vi "Controle_Manip_Main_GUI_WorkingBackup_211222.vi"() -> ()   [LabVIEW 2019] (continued)
                                n1610 = local write "CCD 2D Image Main"(w2024) -> ()
                                }
                                }
                                }
                                }
                              }
                              frame True {
                              }
                            }
                          }
                          frame #1 {
                            # "measurement"
                            n1611 = local read "ESP 301 On?"() -> (w2048:bool)
                            n1612 = case shown="True" w2048 {
                              frame False {
                                n1613 = local read "Log file"() -> (w2052:string)
                                n1614 = call "Write2LogFile.vi"("Add to log file"="ESP301 not activated", "Log file before"=w2052, "Checkbox"=FALSE) -> ("Log file after"=w2051:string)
                                n1615 = local write "Log file"(w2051) -> ()
                              }
                              frame True {
                                n1616 = stacked-sequence {
                                frame #0 {
                                # "get refs and exp params"
                                n1617 = local read "LightField Automation out"() -> (w2063:refnum<class "LightField Automation.lvclass">)
                                n1618 = local read "Photodiode error out"() -> (w2058:errorcluster)
                                n1619 = local read "LightField Automation error out"() -> (w2062:errorcluster)
                                n1620 = local read "ESP 301 COM Port"() -> (w2061:refnum<visa-resource-name>)
                                n1621 = local read "Photodiode handle out"() -> (w2059:refnum<visa-resource-name>)
                                n1622 = local read "ESP 301 Error"() -> (w2060:errorcluster)
                                n1623 = property on="Full scale" class="Bool (strict)"("Val(Sgnl)"=TRUE ("Value (Signaling)")) -> ()  [unwired: 2 in, 2 out]
                                n1624 = Bundle("LightField Automation out"=w2063, "LightField Automation error out"=w2062, "ESP 301 COM Port"=w2061, "ESP 301 Error"=w2060, "Photodiode handle out"=w2059, "Photodiode error out"=w2058) -> (→"Test Handles Polar":T16)  [unwired: 1 in]
                                n1625 = local read "CCD ROI"() -> (w2054:T20)
                                n1626 = local read "Exposure Time (ms)"() -> (w2065:dbl)
                                n1627 = local read "Polar Start Angle (°)"() -> (w2069:dbl)
                                n1628 = local read "Polar Step Angle (°)"() -> (w2068:dbl)
                                n1629 = local read "Polar End Angle (°)"() -> (w2064:dbl)
                                n1630 = local read "KCube Shutter On?"() -> (w2057:bool)
                                n1631 = local read "Polar mode"() -> (w2066:u16)
                                n1632 = local read "Acq Mode"() -> (w2067:T3)
                                n1633 = Bundle("Polar End Angle (°)"=w2064, "Polar Start Angle (°)"=w2069, "Polar Step Angle (°)"=w2068, "Acq Mode"=w2067, "Polar mode"=w2066, "Exposure Time (ms)"=w2065, "CCD ROI"=w2054, "KCube Shutter On?"=w2057) -> (→"Polar Params SubVIv2":T15)  [unwired: 1 in]
                                }
                                frame #1 {
                                # "Prepare graph and controls"
                                n1634 = local read "Scan Polarisation References"() -> (w2073:T17)
                                n1635 = local read "Polar Params SubVIv2"() -> (w2074:T15)
                                n1636 = local read "Scan Polar Params"() -> (w2075:refnum<vi>[])
                                n1637 = call "SubVI_PrePolarisation.vi"("Test References"=w2073, "Polar Params SubVIv2"=w2074, "Scan Polar Params"=w2075) -> ()
                                n1638 = property on="Elapsed (s)" class="DigNum (strict)"("Visible"=TRUE) -> ()  [unwired: 2 in, 2 out]
                                n1639 = property on="CCD 1D Spectrum Main" class="XYGraph (strict)"() -> ("XScale.Maximum"=w2078:dbl, "XScale.Minimum"=w2077:dbl, "YScale.Minimum"=w2072:dbl, "YScale.Maximum"=w2076:dbl)  [unwired: 2 in, 2 out]
                                n1640 = property on="Experiment Graph Controls" class="TabCtl (strict)"("Value"=T25."Polar" ("Experiment Graph Controls")) -> ()  [unwired: 2 in, 2 out]
                                n1641 = property on="Polarisation 1D Spectrum" class="XYGraph (strict)"("XScale.Maximum"=w2078, "XScale.Minimum"=w2077, "YScale.Minimum"=w2072, "YScale.Maximum"=w2076) -> ()  [unwired: 2 in, 2 out]
                                }
                                frame #2 {
                                # "actual exp"
                                n1642 = local read "Scan Polarisation References"() -> (w2085:T17)
                                n1643 = local read "Polar Params SubVIv2"() -> (w2086:T15)
                                n1644 = local read "Test Handles Polar"() -> (w2084:T16)
                                n1645 = call "Polarisation_v2.vi"("Test Handles Polar"=w2084, "Polar Params SubVIv2"=w2086, "Test References"=w2085) -> ("2D Pol Data"=w2083:dbl[][], "Test Handles Out"=w2081:T35, "Angles"=w2082:dbl[], "Wavelengths"=w2079:dbl[], "Puissances"=→"PuissancesPolar":dbl[])  [unwired: 1 in]
                                n1646 = local write "Test Handles Polar"(w2081) -> ()
                                n1647 = local write "Angles"(w2082) -> ()
                                n1648 = local write "Wavelength calibration"(w2079) -> ()
                                n1649 = local write "Pol 2D Array Out"(w2083) -> ()
                                }
                                frame #3 {
                                n1650 = control-ref of="MasterStop"() -> (w2088:refnum<vi>)
                                n1651 = control-ref of="MasterPause"() -> (w2089:refnum<vi>)
                                n1652 = control-ref of="ExperimentStopped?"() -> (w2087:refnum<vi>)
                                n1653 = call "CheckStopAndReset.vi"("ExperimentStopped?"=w2087, "MasterStop"=w2088, "MasterPause"=w2089) -> ()
                                }
                                frame #4 {
                                # "end exp"
                                n1654 = local read "Scan Polarisation References"() -> (w2095:T17)
                                n1655 = local read "Scan Polar Params"() -> (w2096:refnum<vi>[])
                                n1656 = local read "Angles"() -> (w2097:dbl[])
                                n1657 = local read "Test Handles Polar"() -> (w2094:T16)
                                n1658 = call "SubVI_PostPolarisation.vi"("Test References"=w2095, "Angles"=w2097, "Scan Polar Params"=w2096) -> ()
                                n1659 = Unbundle By Name(w2094) -> ("LightField Automation out"=w2093:refnum<class "LightField Automation.lvclass">, "LightField Automation error out"=w2092:errorcluster)
                                n1660 = property on="Elapsed (s)" class="DigNum (strict)"("Visible"=FALSE) -> ()  [unwired: 2 in, 2 out]
                                n1661 = local write "LightField Automation error out"(w2092) -> ()
                                n1662 = local write "LightField Automation out"(w2093) -> ()
                                n1663 = property on="Experiment Graph Controls" class="TabCtl (strict)"("Value"=T25."Polar" ("Experiment Graph Controls")) -> ()  [unwired: 2 in, 2 out]
                                }
                                }
                              }
                            }
                          }
                        }
                      }
                      frame "Acquire Contrast" {
                        n1664 = stacked-sequence {
                          frame #0 {
                            # "background"
                            n1665 = local read "Background taken?"() -> (w2098:bool)
                            n1666 = case shown="False" w2098 {
                              frame False {
                                n1667 = stacked-sequence {
                                tunnel: [_ _ w2148] -> w2099
                                frame #0 {
                                n1668 = local read "Log file"() -> (w2133:string)
                                n1669 = property on="CCD 1D Spectrum Main" class="XYGraph (strict)"("YScale.Offset"=0.0 ("Y Scale.Offset and Multiplier:Offset")) -> ()  [unwired: 2 in, 2 out]
                                n1670 = call "Write2LogFile.vi"("Add to log file"="Acquiring background", "Log file before"=w2133, "Checkbox"=FALSE) -> ("Log file after"=w2132:string)
                                n1671 = local write "Log file"(w2132) -> ()
                                }
                                frame #1 {
                                # "make sure shutter is closed"
                                n1672 = local read "KCube Shutter On?"() -> (w2134:bool)
                                n1673 = control-ref of="Shutter Ctrls"() -> (w2138:refnum<vi>)
                                n1674 = property class="Ring (strict)"(reference=w2138) -> ("Value"=w2137:u16)  [unwired: 1 in, 2 out]
                                n1675 = control-ref of="KCube Shutter Device Reference"() -> (w2139:refnum<vi>)
                                n1676 = Equal?(x=w2137, y=u16 0) -> (x = y?=w2135:bool)
                                n1677 = case shown="False" w2135 {
                                tunnel: w2139 -> [w2142 _]
                                tunnel: w2138 -> [w2141 _]
                                tunnel: w2134 -> [w2140 _]
                                frame False {
                                n1678 = call "Shutter.vi"("KCube Shutter Device Reference 2"=w2142, "Shutter Ctrls 2"=w2141, "Shutter on?"=w2140) -> ()
                                }
                                frame True {
                                }
                                }
                                }
                                frame #2 {
                                # "acquire"
                                n1679 = local read "LightField Automation error out"() -> (w2146:errorcluster)
                                n1680 = local read "LightField Automation out"() -> (w2147:refnum<class "LightField Automation.lvclass">)
                                n1681 = local read "Accumulations"() -> (w2143:dbl)
                                n1682 = call "LFA_Capture.vi"("error in (no error)"=w2146, "Frames"=w2143, "LightField Automation in"=w2147) -> ("error out"=w2145:errorcluster, "Data"=w2148:T26, "LightField Automation out"=w2144:refnum<class "LightField Automation.lvclass">)  [unwired: 6 in]
                                n1683 = local write "LightField Automation error out"(w2145) -> ()
                                n1684 = local write "LightField Automation out"(w2144) -> ()
                                }
                                }
                                n1685 = local read "Acq Mode"() -> (w2100:T3)
                                n1686 = case shown="\"Spectrum\", Default" w2100 {
                                selector: w2100 -> [w2101 w2119]
                                tunnel: w2099 -> [w2102 w2120]
                                frame "Spectrum", Default {
                                n1687 = stacked-sequence {
                                tunnel: w2102 -> [_ w2113 _ _]
                                tunnel: w2101 -> [_ w2111 _ _]
                                frame #0 {
                                n1688 = property on="CCD 2D Image Main" class="IntGraph (strict)"("Visible"=FALSE) -> ()  [unwired: 2 in, 2 out]
                                n1689 = property on="CCD 1D Spectrum Main" class="XYGraph (strict)"("Visible"=TRUE) -> ()  [unwired: 2 in, 2 out]
                                }
                                frame #1 {
                                n1690 = local read "Wavelength calibration"() -> (w2110:dbl[])
                                n1691 = local read "CCD ROI"() -> (w2106:T20)
                                n1692 = Divide(x=1239.842, y=w2110) -> (x/y=w2108:dbl[])
                                n1693 = call "PrepareData4Graph.vi"("Wavelength nm"=w2108, "DataLF"=w2113, "CCD ROI"=w2106, "AcqMode"=w2111, "Data type"=T30."Spectre") -> ("Spectrum"=w2112:cluster{"Array 2":dbl[], "Array":dbl[]}, "PLInt out"=w2105:dbl[])  [unwired: 2 in, 2 out]
                                n1694 = local write "CCD 1D Spectrum Main"(w2112) -> ()
                                n1695 = local write "BackgroundSpec"(w2105) -> ()
                                }
                                frame #2 {
                                n1696 = local read "BackgroundSpec"() -> (w2114:dbl[])
                                n1697 = call-poly <vilib>:"Mean.vi"("X"=w2114) -> ("mean"=w2116:dbl)  [unwired: 1 out]
                                n1698 = Negate(x=w2116) -> (-x=w2115:dbl)
                                n1699 = property on="CCD 1D Spectrum Main" class="XYGraph (strict)"("YScale.Offset"=w2115) -> ()  [unwired: 2 in, 2 out]
                                }
                                frame #3 {
                                n1700 = local write "Background taken?"(TRUE ("Background taken?")) -> ()
                                n1701 = property on="Background substract" class="Enum (strict)"("Value"=enum16{"None", "Shutter"}."None" ("Background substract")) -> ()  [unwired: 2 in, 2 out]
                                }
                                }
                                }
                                frame "Image" {
                                n1702 = stacked-sequence {
                                tunnel: w2120 -> [_ w2128]
                                tunnel: w2119 -> [_ w2126]
                                frame #0 {
                                n1703 = property on="CCD 1D Spectrum Main" class="XYGraph (strict)"("Visible"=FALSE) -> ()  [unwired: 2 in, 2 out]
                                n1704 = property on="CCD 2D Image Main" class="IntGraph (strict)"("Visible"=TRUE) -> ()  [unwired: 2 in, 2 out]
                                }
                                frame #1 {
                                n1705 = local read "Wavelength calibration"() -> (w2127:dbl[])
                                n1706 = local read "CCD ROI"() -> (w2123:T20)
                                n1707 = call "PrepareData4Graph.vi"("Wavelength nm"=w2127, "DataLF"=w2128, "CCD ROI"=w2123, "AcqMode"=w2126, "Data type"=T30."Spectre") -> ("Intensity Graph"=w2125:dbl[][])  [unwired: 2 in, 3 out]
                                n1708 = local write "CCD 2D Image Main"(w2125) -> ()
                                }
                                }
                                }
                                }
                              }
                              frame True {
                              }
                            }
                          }
                          frame #1 {
                            # "measurement"
                            n1709 = stacked-sequence {
                              frame #0 {
                                w2151 = FALSE ("Value")
                                w2152 = TRUE ("Visible")
                                w2156 = FALSE
                                w2161 = FALSE ("Acq Cont")
                                n1710 = property on="CCD 1D Spectrum Main" class="XYGraph (strict)"() -> ("XScale.Maximum"=w2160:dbl, "XScale.Minimum"=w2159:dbl, "YScale.Minimum"=w2158:dbl, "YScale.Maximum"=w2157:dbl)  [unwired: 2 in, 2 out]
                                n1711 = property on="Acquire Contrast" class="Bool (strict)"("Visible"=w2156) -> ()  [unwired: 2 in, 2 out]
                                n1712 = property on="Save Contrast" class="Bool (strict)"("Visible"=w2156) -> ()  [unwired: 2 in, 2 out]
                                n1713 = property on="Contrast 1D Spectrum" class="XYGraph (strict)"("XScale.Maximum"=w2160, "XScale.Minimum"=w2159, "YScale.Minimum"=w2158, "YScale.Maximum"=w2157) -> ()  [unwired: 2 in, 2 out]
                                n1714 = local read "Scan Contrast Ctrls"() -> (w2164:refnum<vi>[])
                                n1715 = property on="Scan Linear Stage Progess Bar" class="Slide (strict)"("Visible"=TRUE, "Value"=u8 0 ("Scan Linear Stage Progess Bar")) -> ()  [unwired: 2 in, 2 out]
                                n1716 = local write "Acquire Contrast"(w2161) -> ()
                                n1717 = local write "Save Contrast"(w2161) -> ()
                                n1718 = call "Enable&Disable_Controls.vi"("Enum"=enum16{"Enabled", "Disabled", "Disabled&Grayed"}."Disabled&Grayed", "References"=w2164) -> ()  [unwired: 1 in]
                                n1719 = property on="Scan Linear Stage Progess Bar" class="Slide (strict)"("Visible"=TRUE) -> ()  [unwired: 2 in, 2 out]
                                n1720 = property on="Elapsed (s)" class="DigNum (strict)"("Visible"=TRUE) -> ()  [unwired: 2 in, 2 out]
                                n1721 = control-ref of="MasterStop"() -> (w2154:refnum<vi>)
                                n1722 = control-ref of="MasterPause"() -> (w2153:refnum<vi>)
                                n1723 = property on="Experiment Graph Controls" class="TabCtl (strict)"("Value"=T25."Contrast" ("Experiment Graph Controls")) -> ()  [unwired: 2 in, 2 out]
                                n1724 = property class="Bool (strict)"(reference=w2153, "Visible"=w2152, "Value"=w2151) -> ()  [unwired: 1 in, 2 out]
                                n1725 = property class="Bool (strict)"(reference=w2154, "Visible"=w2152, "Value"=w2151) -> ()  [unwired: 1 in, 2 out]
                              }
                              frame #1 {
                                n1726 = local read "Excitation Wavelength (nm)"() -> (w2170:dbl)
                                n1727 = local read "LinTFines Step Pos (usteps)"() -> (w2175:dbl)
                                n1728 = local read "LinTFine Start Pos (usteps)"() -> (w2176:dbl)
                                n1729 = local read "LinTFine End Pos (usteps)"() -> (w2174:dbl)
                                n1730 = local read "Exposure Time (ms)"() -> (w2172:dbl)
                                n1731 = local read "LinT Start Pos (mm)"() -> (w2179:dbl)
                                n1732 = local read "LinT Step Pos (mm)"() -> (w2178:dbl)
                                n1733 = local read "LinT End pos (mm)"() -> (w2177:dbl)
                                n1734 = local read "KCube Shutter On?"() -> (w2167:bool)
                                n1735 = local read "Accumulations"() -> (w2171:dbl)
                                n1736 = local read "Acq Mode"() -> (w2169:T3)
                                n1737 = local read "CCD ROI"() -> (w2168:T20)
                                n1738 = Bundle("LinT Start Pos (mm)"=w2179, "LinT Step Pos (mm)"=w2178, "LinT End pos (mm)"=w2177, "LinTFine Start Pos (usteps)"=w2176, "LinTFines Step Pos (usteps)"=w2175, "LinTFine End Pos (usteps)"=w2174) -> (w2173:T27)  [unwired: 1 in]
                                n1739 = Bundle("Exposure Time (ms)"=w2172, "Accumulations"=w2171, "Excitation Wavelength (nm)"=w2170, "Acq Mode"=w2169, "CCD ROI"=w2168, "KCube Shutter On?"=w2167) -> (w2166:T24)  [unwired: 1 in]
                                n1740 = local write "Scan Translation Params"(w2173) -> ()
                                n1741 = local write "Scan Translation Exp Params"(w2166) -> ()
                              }
                              frame #2 {
                                n1742 = local read "Scan Translation Exp Params"() -> (w2187:T24)
                                n1743 = local read "Scan Translation Params"() -> (w2204:T27)
                                n1744 = control-ref of="Scan Linear Stage Progess Bar"() -> ()  [unwired: 1 out]
                                n1745 = control-ref of="Stop Contrast"() -> ()  [unwired: 1 out]
                                n1746 = local read "ESP 301 COM Port"() -> (w2197:refnum<visa-resource-name>)
                                n1747 = control-ref of="Pause Contrast"() -> ()  [unwired: 1 out]
                                n1748 = control-ref of="Scan Main Progess Bar"() -> (w2186:refnum<vi>)
                                n1749 = local read "LightField Automation error out"() -> (w2184:errorcluster)
                                n1750 = local read "ESP 301 Error"() -> (w2199:errorcluster)
                                n1751 = local read "LightField Automation out"() -> (w2185:refnum<class "LightField Automation.lvclass">)
                                n1752 = control-ref of="Shutter Ctrls"() -> (w2189:refnum<vi>)
                                n1753 = control-ref of="KCube Shutter Device Reference"() -> (w2190:refnum<vi>)
                                n1754 = control-ref of="PZC Position Readout (usteps)"() -> (w2188:refnum<vi>)
                                n1755 = control-ref of="Contrast 1D Spectrum"() -> (w2191:refnum<vi>)
                                n1756 = control-ref of="Contrast Oscillations"() -> (w2192:refnum<vi>)
                                n1757 = Open VI Reference(type specifier VI Refnum (for type only)=refnum<vi> refnum ("application reference (local)"), vi path=path "C:/Users/manip/Documents/Controle_Manip_2020/subVIs/Scans/FineContrast_cleaned inputs.vi", options=256) -> (vi reference=w2202:refnum<vi>, error out=w2211:errorcluster)  [unwired: 3 in]
                                n1758 = local read "PZC200 Instrument Channel"() -> (w2203:string)
                                n1759 = call-by-ref "Wait On Asynchronous Call"(reference=w2202, error in=w2211) -> (reference out=w2210:refnum<vi>, error out=w2209:errorcluster, "PZAPos & InstPow"=w2200:dbl[][], "Spectra vs PZA"=w2207:i32[][], "LFA out"=w2183:refnum<class "LightField Automation.lvclass">, "PZC out"=w2201:string, "Photodiode out"=w2193:refnum<visa-resource-name>, "ESP 301 COM out"=w2196:refnum<visa-resource-name>, "LFA error out"=w2182:errorcluster, "PZC error out"=w2194:errorcluster, "Photodiode error out"=w2195:errorcluster, "ESP 301 error out"=w2198:errorcluster)  [unwired: 18 in]
                                n1760 = local write "PZAPos&Pow"(w2200) -> ()
                                n1761 = local write "Photodiode error out"(w2195) -> ()
                                n1762 = local write "PZC200 Instrument Channel"(w2201) -> ()
                                n1763 = local write "Contrast Array Out"(w2207) -> ()
                                n1764 = local read "PZC Error"() -> (w2208:errorcluster)
                                n1765 = local write "ESP 301 COM Port"(w2196) -> ()
                                n1766 = Close Reference(reference=w2210, error in (no error)=w2209) -> ()  [unwired: 1 out]
                                n1767 = local write "Photodiode handle out"(w2193) -> ()
                                n1768 = local read "Photodiode handle out"() -> (w2205:refnum<visa-resource-name>)
                                n1769 = local write "ESP 301 Error"(w2198) -> ()
                                n1770 = local read "Photodiode error out"() -> (w2206:errorcluster)
                                n1771 = local write "LightField Automation error out"(w2182) -> ()
                                n1772 = local write "LightField Automation out"(w2183) -> ()
                                n1773 = local write "PZC Error"(w2194) -> ()
                                n1774 = control-ref of="MasterStop"() -> (w2180:refnum<vi>)
                                n1775 = control-ref of="MasterPause"() -> (w2181:refnum<vi>)
                                n1776 = call-by-ref "Start Asynchronous Call"(reference=w2202, error in=w2211, "LFA in"=w2185, "PZC in"=w2203, "Photodiode in"=w2205, "ESP 301 COM"=w2197, "LFA error in"=w2184, "PZC error in"=w2208, "Photodiode error in"=w2206, "ESP 301 error in"=w2199, "Scan Translation Exp Params"=w2187, "PZC Pos (usteps)"=w2188, "Scan Translation Params"=w2204, "Pause button"=w2181, "Contrast Oscillations"=w2192, "Stop button"=w2180, "Contrast 1D Spectrum"=w2191, "Progess Bar"=w2186, "Shutter Device"=w2190, "Shutter"=w2189) -> ()  [unwired: 12 out]
                              }
                              frame #3 {
                                w2227 = FALSE ("Acq Cont")
                                w2224 = FALSE ("Acq Cont")
                                n1777 = local read "Auto< ?"() -> (w2222:bool)
                                n1778 = property on="Scan Linear Stage Progess Bar" class="Slide (strict)"("Visible"=FALSE, "Value"=u8 0 ("Scan Linear Stage Progess Bar")) -> ()  [unwired: 2 in, 2 out]
                                n1779 = Not(x=w2222) -> (.not. x?=w2221:bool)
                                n1780 = local write "Pause Michelson"(w2227) -> ()
                                n1781 = local write "Stop Michelson"(w2227) -> ()
                                n1782 = property on="Save Contrast" class="Bool (strict)"("Visible"=w2221) -> ()  [unwired: 2 in, 2 out]
                                n1783 = property on="Acquire Contrast" class="Bool (strict)"("Visible"=TRUE) -> ()  [unwired: 2 in, 2 out]
                                n1784 = local write "Acquire Michelson"(w2224) -> ()
                                n1785 = local write "Acquire Contrast"(w2224) -> ()
                                n1786 = local write "Save Michelson"(w2224) -> ()
                                n1787 = local read "Scan Contrast Ctrls"() -> (w2220:refnum<vi>[])
                                n1788 = property on="Elapsed (s)" class="DigNum (strict)"("Visible"=FALSE) -> ()  [unwired: 2 in, 2 out]
                                n1789 = control-ref of="MasterStop"() -> (w2217:refnum<vi>)
                                n1790 = control-ref of="MasterPause"() -> (w2218:refnum<vi>)
                                n1791 = call "Enable&Disable_Controls.vi"("Enum"=enum16{"Enabled", "Disabled", "Disabled&Grayed"}."Enabled", "References"=w2220) -> ()  [unwired: 1 in]
                                n1792 = control-ref of="ExperimentStopped?"() -> (w2216:refnum<vi>)
                                n1793 = call "CheckStopAndReset.vi"("ExperimentStopped?"=w2216, "MasterStop"=w2217, "MasterPause"=w2218) -> ()
                              }
                            }
                          }
                        }
                      }
                      frame "Acquire Michelson" {
                        n1794 = stacked-sequence {
                          frame #0 {
                            # "background"
                            n1795 = local read "Background taken?"() -> (w2228:bool)
                            n1796 = case shown="False" w2228 {
                              frame False {
                                n1797 = stacked-sequence {
                                tunnel: [_ _ w2278] -> w2229
                                frame #0 {
                                n1798 = local read "Log file"() -> (w2263:string)
                                n1799 = property on="CCD 1D Spectrum Main" class="XYGraph (strict)"("YScale.Offset"=0.0 ("Y Scale.Offset and Multiplier:Offset")) -> ()  [unwired: 2 in, 2 out]
                                n1800 = call "Write2LogFile.vi"("Add to log file"="Acquiring background", "Log file before"=w2263, "Checkbox"=FALSE) -> ("Log file after"=w2262:string)
                                n1801 = local write "Log file"(w2262) -> ()
                                }
                                frame #1 {
                                # "make sure shutter is closed"
                                n1802 = local read "KCube Shutter On?"() -> (w2264:bool)
                                n1803 = control-ref of="Shutter Ctrls"() -> (w2268:refnum<vi>)
                                n1804 = property class="Ring (strict)"(reference=w2268) -> ("Value"=w2267:u16)  [unwired: 1 in, 2 out]
                                n1805 = control-ref of="KCube Shutter Device Reference"() -> (w2269:refnum<vi>)
                                n1806 = Equal?(x=w2267, y=u16 0) -> (x = y?=w2265:bool)
                                n1807 = case shown="False" w2265 {
                                tunnel: w2269 -> [w2272 _]
                                tunnel: w2268 -> [w2271 _]
                                tunnel: w2264 -> [w2270 _]
                                frame False {
                                n1808 = call "Shutter.vi"("KCube Shutter Device Reference 2"=w2272, "Shutter Ctrls 2"=w2271, "Shutter on?"=w2270) -> ()
                                }
                                frame True {
                                }
                                }
                                }
                                frame #2 {
                                # "acquire"
                                n1809 = local read "LightField Automation error out"() -> (w2276:errorcluster)
                                n1810 = local read "LightField Automation out"() -> (w2277:refnum<class "LightField Automation.lvclass">)
                                n1811 = local read "Accumulations"() -> (w2273:dbl)
                                n1812 = call "LFA_Capture.vi"("error in (no error)"=w2276, "Frames"=w2273, "LightField Automation in"=w2277) -> ("error out"=w2275:errorcluster, "Data"=w2278:T26, "LightField Automation out"=w2274:refnum<class "LightField Automation.lvclass">)  [unwired: 6 in]
                                n1813 = local write "LightField Automation error out"(w2275) -> ()
                                n1814 = local write "LightField Automation out"(w2274) -> ()
                                }
                                }
                                n1815 = local read "Acq Mode"() -> (w2230:T3)
                                n1816 = case shown="\"Spectrum\", Default" w2230 {
                                selector: w2230 -> [w2231 w2249]
                                tunnel: w2229 -> [w2232 w2250]
                                frame "Spectrum", Default {
                                n1817 = stacked-sequence {
                                tunnel: w2232 -> [_ w2243 _ _]
                                tunnel: w2231 -> [_ w2241 _ _]
                                frame #0 {
                                n1818 = property on="CCD 2D Image Main" class="IntGraph (strict)"("Visible"=FALSE) -> ()  [unwired: 2 in, 2 out]
                                n1819 = property on="CCD 1D Spectrum Main" class="XYGraph (strict)"("Visible"=TRUE) -> ()  [unwired: 2 in, 2 out]
                                }
                                frame #1 {
                                n1820 = local read "Wavelength calibration"() -> (w2240:dbl[])
                                n1821 = local read "CCD ROI"() -> (w2236:T20)
                                n1822 = Divide(x=1239.842, y=w2240) -> (x/y=w2238:dbl[])
                                n1823 = call "PrepareData4Graph.vi"("Wavelength nm"=w2238, "DataLF"=w2243, "CCD ROI"=w2236, "AcqMode"=w2241, "Data type"=T30."Spectre") -> ("Spectrum"=w2242:cluster{"Array 2":dbl[], "Array":dbl[]}, "PLInt out"=w2235:dbl[])  [unwired: 2 in, 2 out]
                                n1824 = local write "CCD 1D Spectrum Main"(w2242) -> ()
                                n1825 = local write "BackgroundSpec"(w2235) -> ()
                                }
                                frame #2 {
                                n1826 = local read "BackgroundSpec"() -> (w2244:dbl[])
                                n1827 = call-poly <vilib>:"Mean.vi"("X"=w2244) -> ("mean"=w2246:dbl)  [unwired: 1 out]
                                n1828 = Negate(x=w2246) -> (-x=w2245:dbl)
                                n1829 = property on="CCD 1D Spectrum Main" class="XYGraph (strict)"("YScale.Offset"=w2245) -> ()  [unwired: 2 in, 2 out]
                                }
                                frame #3 {
                                n1830 = local write "Background taken?"(TRUE ("Background taken?")) -> ()
                                n1831 = property on="Background substract" class="Enum (strict)"("Value"=enum16{"None", "Shutter"}."None" ("Background substract")) -> ()  [unwired: 2 in, 2 out]
                                }
                                }
                                }
                                frame "Image" {
                                n1832 = stacked-sequence {
                                tunnel: w2250 -> [_ w2258]
                                tunnel: w2249 -> [_ w2256]
                                frame #0 {
                                n1833 = property on="CCD 1D Spectrum Main" class="XYGraph (strict)"("Visible"=FALSE) -> ()  [unwired: 2 in, 2 out]
                                n1834 = property on="CCD 2D Image Main" class="IntGraph (strict)"("Visible"=TRUE) -> ()  [unwired: 2 in, 2 out]
                                }
                                frame #1 {
                                n1835 = local read "Wavelength calibration"() -> (w2257:dbl[])
                                n1836 = local read "CCD ROI"() -> (w2253:T20)
                                n1837 = call "PrepareData4Graph.vi"("Wavelength nm"=w2257, "DataLF"=w2258, "CCD ROI"=w2253, "AcqMode"=w2256, "Data type"=T30."Spectre") -> ("Intensity Graph"=w2255:dbl[][])  [unwired: 2 in, 3 out]
                                n1838 = local write "CCD 2D Image Main"(w2255) -> ()
                                }
                                }
                                }
                                }
                              }
                              frame True {
                              }
                            }
                          }
                          frame #1 {
                            # "measurement"
                            n1839 = Get Date/Time In Seconds() -> (seconds since 1Jan1904=w2279:timestamp)
                            n1840 = stacked-sequence {
                              tunnel: w2279 -> [_ _ w2313 w2437]
                              frame #0 {
                                w2285 = TRUE
                                w2286 = FALSE ("Acq Cont")
                                w2283 = TRUE
                                w2282 = FALSE
                                w2284 = FALSE
                                # "check that range is within translation stage travel"
                                # "get params and check feasability"
                                n1841 = property on="Save Michelson" class="Bool (strict)"("Visible"=w2284) -> ()  [unwired: 2 in, 2 out]
                                n1842 = property on="Pause Michelson" class="Bool (strict)"("Visible"=w2283) -> ()  [unwired: 2 in, 2 out]
                                n1843 = property on="Save Contrast" class="Bool (strict)"("Visible"=w2284) -> ()  [unwired: 2 in, 2 out]
                                n1844 = property on="Pause Contrast" class="Bool (strict)"("Visible"=w2283) -> ()  [unwired: 2 in, 2 out]
                                n1845 = property on="Stop Contrast" class="Bool (strict)"("Visible"=w2283) -> ()  [unwired: 2 in, 2 out]
                                n1846 = property on="Acquire Michelson" class="Bool (strict)"("Visible"=w2284) -> ()  [unwired: 2 in, 2 out]
                                n1847 = property on="Stop Michelson" class="Bool (strict)"("Visible"=w2283) -> ()  [unwired: 2 in, 2 out]
                                n1848 = property on="Acquire Contrast" class="Bool (strict)"("Visible"=w2284) -> ()  [unwired: 2 in, 2 out]
                                n1849 = property on="Scan Linear Stage Progess Bar" class="Slide (strict)"("Visible"=TRUE, "Value"=u8 0 ("Scan Linear Stage Progess Bar")) -> ()  [unwired: 2 in, 2 out]
                                n1850 = property on="Scan Michelson Progess Bar" class="Slide (strict)"("Value"=u8 0 ("Scan Michelson Progess Bar"), "Visible"=TRUE) -> ()  [unwired: 2 in, 2 out]
                                n1851 = local read "Scan Contrast Ctrls"() -> (w2292:refnum<vi>[])
                                n1852 = local write "Acquire Contrast"(w2286) -> ()
                                n1853 = local write "Save Contrast"(w2286) -> ()
                                n1854 = call "Enable&Disable_Controls.vi"("Enum"=enum16{"Enabled", "Disabled", "Disabled&Grayed"}."Disabled&Grayed", "References"=w2292) -> ()  [unwired: 1 in]
                                n1855 = property on="Michelson Expected (s)" class="DigNum (strict)"("Visible"=w2285) -> ()  [unwired: 2 in, 2 out]
                                n1856 = property on="Elapsed (s)" class="DigNum (strict)"("Visible"=TRUE) -> ()  [unwired: 2 in, 2 out]
                                n1857 = property on="Experiment Graph Controls" class="TabCtl (strict)"("Value"=T25."Contrast" ("Experiment Graph Controls")) -> ()  [unwired: 2 in, 2 out]
                                n1858 = property on="Michelson Elapsed (s)" class="DigNum (strict)"("Visible"=w2285) -> ()  [unwired: 2 in, 2 out]
                                n1859 = local write "Acquire Michelson"(w2282) -> ()
                                n1860 = local write "Save Michelson"(w2282) -> ()
                              }
                              frame #1 {
                                # "check that range is within translation stage travel"
                                # "get params"
                                n1861 = local read "Excitation Wavelength (nm)"() -> (w2297:dbl)
                                n1862 = local read "Exposure Time (ms)"() -> (w2299:dbl)
                                n1863 = local read "KCube Shutter On?"() -> (w2294:bool)
                                n1864 = local read "Accumulations"() -> (w2298:dbl)
                                n1865 = local read "Acq Mode"() -> (w2296:T3)
                                n1866 = local read "CCD ROI"() -> (w2295:T20)
                                n1867 = local read "LinTFines Step Pos (usteps)"() -> (w2302:dbl)
                                n1868 = local read "LinTFine Start Pos (usteps)"() -> (w2303:dbl)
                                n1869 = local read "LinTFine End Pos (usteps)"() -> (w2301:dbl)
                                n1870 = local read "LinT Start Pos (mm)"() -> (w2306:dbl)
                                n1871 = local read "LinT Step Pos (mm)"() -> (w2305:dbl)
                                n1872 = local read "LinT End pos (mm)"() -> (w2304:dbl)
                                n1873 = Bundle("Exposure Time (ms)"=w2299, "Accumulations"=w2298, "Excitation Wavelength (nm)"=w2297, "Acq Mode"=w2296, "CCD ROI"=w2295, "KCube Shutter On?"=w2294) -> (w2293:T24)  [unwired: 1 in]
                                n1874 = Bundle("LinT Start Pos (mm)"=w2306, "LinT Step Pos (mm)"=w2305, "LinT End pos (mm)"=w2304, "LinTFine Start Pos (usteps)"=w2303, "LinTFines Step Pos (usteps)"=w2302, "LinTFine End Pos (usteps)"=w2301) -> (w2300:T27)  [unwired: 1 in]
                                n1875 = local write "Scan Translation Exp Params"(w2293) -> ()
                                n1876 = local write "Scan Translation Params"(w2300) -> ()
                              }
                              frame #2 {
                                # "pzc & inst pow"
                                # "esp pos"
                                # "data"
                                # "move ESP"
                                n1877 = local read "LightField Automation out"() -> (w2310:refnum<class "LightField Automation.lvclass">)
                                n1878 = local read "ESP 301 COM Port"() -> (w2312:refnum<visa-resource-name>)
                                n1879 = local read "LinT Start Pos (mm)"() -> (w2323:dbl)
                                n1880 = local read "ESP 301 Error"() -> (w2319:errorcluster)
                                n1881 = local read "LinT Step Pos (mm)"() -> (w2324:dbl)
                                n1882 = local read "LinT End pos (mm)"() -> (w2328:dbl)
                                n1883 = local read "LinT Start Pos (mm)"() -> (w2329:dbl)
                                n1884 = local read "LinT Step Pos (mm)"() -> (w2326:dbl)
                                n1885 = local read "LightField Automation error out"() -> (w2309:errorcluster)
                                n1886 = Subtract(x=w2328, y=w2329) -> (x-y=w2327:dbl)
                                n1887 = Divide(x=w2327, y=w2326) -> (x/y=w2325:dbl)
                                n1888 = Increment(x=w2325) -> (x+1=w2322:dbl)
                                n1889 = for {
                                N: w2322 -> [w2335]
                                tunnel: w2324 -> [w2352]
                                tunnel: w2323 -> [w2351]
                                shift-right: [w2347] -> w2320
                                shift-left: dbl[] [] -> [w2348]
                                shift-right: [w2345] -> w2308
                                shift-left: w2310 -> [w2346]
                                shift-right: [w2343] -> w2307
                                shift-left: w2309 -> [w2344]
                                shift-right: [w2341] -> w2318
                                shift-left: w2319 -> [w2342]
                                shift-right: [w2339] -> w2316
                                shift-left: dbl[][][] [] -> [w2340]
                                shift-right: [w2337] -> w2314
                                shift-left: dbl[][][] [] -> [w2338]
                                tunnel: w2313 -> [w2333]
                                shift-right: [w2330] -> w2311
                                shift-left: w2312 -> [w2331]
                                i -> [w2334]
                                stop <- w2332 stop-if-true
                                # "ESP"
                                n1890 = Multiply(x=w2334, y=w2352) -> (x*y=w2350:dbl)
                                n1891 = Add(x=w2351, y=w2350) -> (x+y=w2349:dbl)
                                n1892 = Divide(x=w2334, y=w2335) -> (x/y=w2336:dbl)
                                n1893 = stacked-sequence {
                                tunnel: w2349 -> [w2357 w2363 _ _]
                                tunnel: w2348 -> [w2359 _ _ _]
                                tunnel: [w2358 _ _ _] -> w2347
                                tunnel: w2346 -> [_ _ w2406 _]
                                tunnel: [_ _ w2405 _] -> w2345
                                tunnel: w2344 -> [_ _ w2404 _]
                                tunnel: [_ _ w2403 _] -> w2343
                                tunnel: w2342 -> [w2356 _ _ _]
                                tunnel: [w2355 _ _ _] -> w2341
                                tunnel: w2340 -> [_ _ w2375 _]
                                tunnel: [_ _ w2373 _] -> w2339
                                tunnel: w2338 -> [_ _ w2372 _]
                                tunnel: [_ _ w2370 _] -> w2337
                                tunnel: w2336 -> [_ _ _ w2416]
                                tunnel: w2335 -> [_ _ _ w2415]
                                tunnel: w2334 -> [_ _ _ w2413]
                                tunnel: w2333 -> [_ _ _ w2414]
                                tunnel: [_ _ _ w2411] -> w2332
                                tunnel: w2331 -> [w2354 _ _ _]
                                tunnel: [w2353 _ _ _] -> w2330
                                frame #0 {
                                # "pos readout"
                                n1894 = control-ref of="Newport Linear Translation Stage Position Readout (mm)"() -> (w2360:refnum<vi>)
                                n1895 = call "ESP301_Go2Pos.vi"("VISA resource name"=w2354, "Set value"=w2357, "Axis (1)"=1, "Error In"=w2356, "DigNum Refnum"=w2360) -> ("VISA resource name 2"=w2353:refnum<visa-resource-name>, "Error In 2"=w2355:errorcluster)
                                n1896 = Insert Into Array(array=w2359, new element=w2357) -> (w2358:dbl[])  [unwired: 1 in]
                                }
                                frame #1 {
                                # "wait on ESP"
                                n1897 = Wait (ms)(milliseconds to wait=u32 50) -> ()  [unwired: 1 out]
                                n1898 = Number To Decimal String(number=w2363) -> (decimal integer string=w2366:string)  [unwired: 1 in]
                                n1899 = local read "Log file"() -> (w2369:string)
                                n1900 = Concatenate Strings("ESP moved to ", w2366) -> (w2365:string)
                                n1901 = call "Write2LogFile.vi"("Add to log file"=w2365, "Log file before"=w2369, "Checkbox"=FALSE) -> ("Log file after"=w2368:string)
                                n1902 = local write "Log file"(w2368) -> ()
                                }
                                frame #2 {
                                n1903 = control-ref of="Shutter Ctrls"() -> (w2393:refnum<vi>)
                                n1904 = control-ref of="Scan Linear Stage Progess Bar"() -> (w2389:refnum<vi>)
                                n1905 = control-ref of="KCube Shutter Device Reference"() -> (w2394:refnum<vi>)
                                n1906 = control-ref of="PZC Position Readout (usteps)"() -> (w2392:refnum<vi>)
                                n1907 = control-ref of="Pause Contrast"() -> (w2391:refnum<vi>)
                                n1908 = control-ref of="Contrast 1D Spectrum"() -> (w2395:refnum<vi>)
                                n1909 = control-ref of="Contrast Oscillations"() -> (w2396:refnum<vi>)
                                n1910 = local read "Photodiode handle out"() -> (w2385:refnum<visa-resource-name>)
                                n1911 = local read "Photodiode error out"() -> (w2386:errorcluster)
                                n1912 = control-ref of="Stop Contrast"() -> (w2390:refnum<vi>)
                                n1913 = local read "Scan Translation Params"() -> (w2398:T27)
                                n1914 = Open VI Reference(type specifier VI Refnum (for type only)=refnum<vi> refnum ("application reference (local)"), vi path=path "C:/Users/manip/Documents/Controle_Manip_2020/subVIs/Scans/FineContrast_cleaned inputs.vi", options=256) -> (vi reference=w2400:refnum<vi>, error out=w2399:errorcluster)  [unwired: 3 in]
                                n1915 = local read "Scan Translation Exp Params"() -> (w2397:T24)
                                n1916 = local read "PZC200 Instrument Channel"() -> (w2384:string)
                                n1917 = local read "ESP 301 Error"() -> (w2387:errorcluster)
                                n1918 = local read "PZC Error"() -> (w2383:errorcluster)
                                n1919 = local read "ESP 301 COM Port"() -> (w2388:refnum<visa-resource-name>)
                                n1920 = call-by-ref "Start Asynchronous Call"(reference=w2400, error in=w2399, "LFA in"=w2406, "PZC in"=w2384, "Photodiode in"=w2385, "ESP 301 COM"=w2388, "LFA error in"=w2404, "PZC error in"=w2383, "Photodiode error in"=w2386, "ESP 301 error in"=w2387, "Scan Translation Exp Params"=w2397, "PZC Pos (usteps)"=w2392, "Scan Translation Params"=w2398, "Pause button"=w2391, "Contrast Oscillations"=w2396, "Stop button"=w2390, "Contrast 1D Spectrum"=w2395, "Progess Bar"=w2389, "Shutter Device"=w2394, "Shutter"=w2393) -> ()  [unwired: 12 out]
                                n1921 = call-by-ref "Wait On Asynchronous Call"(reference=w2400, error in=w2399) -> ("PZAPos & InstPow"=w2371:dbl[][], "Spectra vs PZA"=w2374:i32[][], "LFA out"=w2405:refnum<class "LightField Automation.lvclass">, "PZC out"=w2380:string, "Photodiode out"=w2379:refnum<visa-resource-name>, "ESP 301 COM out"=w2381:refnum<visa-resource-name>, "LFA error out"=w2403:errorcluster, "PZC error out"=w2377:errorcluster, "Photodiode error out"=w2378:errorcluster, "ESP 301 error out"=w2382:errorcluster)  [unwired: 18 in, 2 out]
                                n1922 = local write "PZC200 Instrument Channel"(w2380) -> ()
                                n1923 = local write "Photodiode handle out"(w2379) -> ()
                                n1924 = local write "Photodiode error out"(w2378) -> ()
                                n1925 = local write "ESP 301 COM Port"(w2381) -> ()
                                n1926 = Insert Into Array(array=w2372, new element=w2371) -> (w2370:dbl[][][])  [unwired: 3 in]
                                n1927 = local write "ESP 301 Error"(w2382) -> ()
                                n1928 = local write "PZC Error"(w2377) -> ()
                                n1929 = Insert Into Array(array=w2375, new element=w2374) -> (w2373:dbl[][][])  [unwired: 3 in]
                                }
                                frame #3 {
                                n1930 = local read "Pause Michelson"() -> (w2410:bool)
                                n1931 = control-ref of="Expected (s)"() -> (w2408:refnum<vi>)
                                n1932 = Increment(x=w2413) -> (x+1=w2412:i32)
                                n1933 = Multiply(x=w2416, y=100.0) -> (x*y=w2418:dbl)
                                n1934 = call "Expectedtime.vi"("N"=w2415, "I"=w2412, "Reference time"=w2414) -> ("Expected time"=w2407:dbl, "Elapsed time"=w2409:dbl)
                                "Michelson Elapsed (s)" <- w2409
                                "Michelson Expected (s)" <- w2407
                                n1935 = property class="DigNum (strict)"(reference=w2408, "Value"=w2407) -> ()  [unwired: 1 in, 2 out]
                                n1936 = property on="Elapsed (s)" class="DigNum (strict)"("Value"=w2409) -> ()  [unwired: 2 in, 2 out]
                                n1937 = local write "Scan Michelson Progess Bar"(w2418) -> ()
                                n1938 = case shown="True" w2410 {
                                frame False {
                                }
                                frame True {
                                n1939 = while {
                                stop <- w2420 stop-if-true
                                n1940 = local read "Pause Michelson"() -> (w2421:bool)
                                n1941 = Wait (ms)(milliseconds to wait=u32 50) -> ()  [unwired: 1 out]
                                n1942 = Not(x=w2421) -> (.not. x?=w2420:bool)
                                }
                                }
                                }
                                n1943 = local read "Stop Michelson"() -> (w2411:bool)
                                }
                                }
                                }
                                "ESP Pos" <- w2320
                                "PZC&Pow3D" <- w2314
                                n1944 = local write "LightField Automation error out"(w2307) -> ()
                                n1945 = local write "LightField Automation out"(w2308) -> ()
                                n1946 = local write "ESP 301 COM Port"(w2311) -> ()
                                n1947 = local write "Michelson Array Out"(w2316) -> ()
                                n1948 = local write "ESP 301 Error"(w2318) -> ()
                              }
                              frame #3 {
                                w2429 = FALSE
                                w2431 = FALSE
                                w2428 = FALSE ("Visible")
                                n1949 = Get Date/Time In Seconds() -> (seconds since 1Jan1904=w2438:timestamp)
                                n1950 = property on="Scan Linear Stage Progess Bar" class="Slide (strict)"("Visible"=FALSE) -> ()  [unwired: 2 in, 2 out]
                                n1951 = Subtract(x=w2438, y=w2437) -> (x-y=w2436:dbl)
                                n1952 = property on="Stop Michelson" class="Bool (strict)"("Visible"=w2429) -> ()  [unwired: 2 in, 2 out]
                                n1953 = property on="Pause Michelson" class="Bool (strict)"("Visible"=w2429) -> ()  [unwired: 2 in, 2 out]
                                n1954 = local write "Michelson Elapsed (s)"(w2436) -> ()
                                n1955 = local read "Auto< ?"() -> (w2427:bool)
                                n1956 = Not(x=w2427) -> (.not. x?=w2426:bool)
                                n1957 = property on="Save Michelson" class="Bool (strict)"("Visible"=w2426) -> ()  [unwired: 2 in, 2 out]
                                n1958 = property on="Acquire Michelson" class="Bool (strict)"("Visible"=TRUE) -> ()  [unwired: 2 in, 2 out]
                                n1959 = property on="Acquire Contrast" class="Bool (strict)"("Visible"=TRUE) -> ()  [unwired: 2 in, 2 out]
                                n1960 = property on="Save Contrast" class="Bool (strict)"("Visible"=w2426) -> ()  [unwired: 2 in, 2 out]
                                n1961 = property on="Pause Contrast" class="Bool (strict)"("Visible"=w2431) -> ()  [unwired: 2 in, 2 out]
                                n1962 = property on="Stop Contrast" class="Bool (strict)"("Visible"=w2431) -> ()  [unwired: 2 in, 2 out]
                                n1963 = property on="Elapsed (s)" class="DigNum (strict)"("Visible"=TRUE) -> ()  [unwired: 2 in, 2 out]
                                n1964 = property on="Michelson Expected (s)" class="DigNum (strict)"("Visible"=w2428) -> ()  [unwired: 2 in, 2 out]
                                n1965 = local read "Scan Contrast Ctrls"() -> (w2435:refnum<vi>[])
                                n1966 = control-ref of="MasterStop"() -> (w2424:refnum<vi>)
                                n1967 = control-ref of="MasterPause"() -> (w2425:refnum<vi>)
                                n1968 = property on="Michelson Elapsed (s)" class="DigNum (strict)"("Visible"=w2428) -> ()  [unwired: 2 in, 2 out]
                                n1969 = property on="Scan Michelson Progess Bar" class="Slide (strict)"("Visible"=w2428) -> ()  [unwired: 2 in, 2 out]
                                n1970 = control-ref of="ExperimentStopped?"() -> (w2423:refnum<vi>)
                                n1971 = call "CheckStopAndReset.vi"("ExperimentStopped?"=w2423, "MasterStop"=w2424, "MasterPause"=w2425) -> ()
                                n1972 = call "Enable&Disable_Controls.vi"("Enum"=enum16{"Enabled", "Disabled", "Disabled&Grayed"}."Enabled", "References"=w2435) -> ()  [unwired: 1 in]
                              }
                            }
                          }
                        }
                      }
                      frame "Acquire XY Map" {
                        n1973 = stacked-sequence {
                          frame #0 {
                            # "background"
                            n1974 = local read "Background taken?"() -> (w2439:bool)
                            n1975 = case shown="False" w2439 {
                              frame False {
                                n1976 = stacked-sequence {
                                tunnel: [_ _ w2489] -> w2440
                                frame #0 {
                                n1977 = local read "Log file"() -> (w2474:string)
                                n1978 = property on="CCD 1D Spectrum Main" class="XYGraph (strict)"("YScale.Offset"=0.0 ("Y Scale.Offset and Multiplier:Offset")) -> ()  [unwired: 2 in, 2 out]
                                n1979 = call "Write2LogFile.vi"("Add to log file"="Acquiring background", "Log file before"=w2474, "Checkbox"=FALSE) -> ("Log file after"=w2473:string)
                                n1980 = local write "Log file"(w2473) -> ()
                                }
                                frame #1 {
                                # "make sure shutter is closed"
                                n1981 = local read "KCube Shutter On?"() -> (w2475:bool)
                                n1982 = control-ref of="Shutter Ctrls"() -> (w2479:refnum<vi>)
                                n1983 = property class="Ring (strict)"(reference=w2479) -> ("Value"=w2478:u16)  [unwired: 1 in, 2 out]
                                n1984 = control-ref of="KCube Shutter Device Reference"() -> (w2480:refnum<vi>)
                                n1985 = Equal?(x=w2478, y=u16 0) -> (x = y?=w2476:bool)
                                n1986 = case shown="False" w2476 {
                                tunnel: w2480 -> [w2483 _]
                                tunnel: w2479 -> [w2482 _]
                                tunnel: w2475 -> [w2481 _]
                                frame False {
                                n1987 = call "Shutter.vi"("KCube Shutter Device Reference 2"=w2483, "Shutter Ctrls 2"=w2482, "Shutter on?"=w2481) -> ()
                                }
                                frame True {
                                }
                                }
                                }
                                frame #2 {
                                # "acquire"
                                n1988 = local read "LightField Automation error out"() -> (w2487:errorcluster)
                                n1989 = local read "LightField Automation out"() -> (w2488:refnum<class "LightField Automation.lvclass">)
                                n1990 = local read "Accumulations"() -> (w2484:dbl)
                                n1991 = call "LFA_Capture.vi"("error in (no error)"=w2487, "Frames"=w2484, "LightField Automation in"=w2488) -> ("error out"=w2486:errorcluster, "Data"=w2489:T26, "LightField Automation out"=w2485:refnum<class "LightField Automation.lvclass">)  [unwired: 6 in]
                                n1992 = local write "LightField Automation error out"(w2486) -> ()
                                n1993 = local write "LightField Automation out"(w2485) -> ()
                                }
                                }
                                n1994 = local read "Acq Mode"() -> (w2441:T3)
                                n1995 = case shown="\"Spectrum\", Default" w2441 {
                                selector: w2441 -> [w2442 w2460]
                                tunnel: w2440 -> [w2443 w2461]
                                frame "Spectrum", Default {
                                n1996 = stacked-sequence {
                                tunnel: w2443 -> [_ w2454 _ _]
                                tunnel: w2442 -> [_ w2452 _ _]